vi "UHR-Fleezers Control (host) - 10.2.vi"() -> ()   [LabVIEW 2009] (continued)
        n1205 = local read "AI2 (V)"() -> (w4676:cluster{"Set 1":dbl, "Set 2":dbl})
        n1206 = Or Array Elements(Boolean array=w4678) -> (logical OR=w4679:bool)
        n1207 = Bundle By Name(cluster=w4676, "Set 1"=w4675, "Set 2"=w4674) -> (w4673:cluster{"Set 1":dbl, "Set 2":dbl})
        n1208 = Divide(x=w4673, y=3276.7) -> (x/y=w4672:cluster{"Set 1":dbl, "Set 2":dbl})
        "AI2 (V)" <- w4672
        n1209 = case shown="True" w4679 {
          tunnel: [w4741 w4758] -> w4671
          tunnel: "AI2 to Setpoint" -> [_ w4754]
          tunnel: "Setpoints (V)" -> [w4742 w4757]
          tunnel: w4672 -> [_ w4751]
          frame #0 {
            n1210 = Multiply(x=3276.7, y=w4742) -> (x*y=w4743:cluster{"Set 1":dbl, "Set 2":dbl})
            n1211 = To Word Integer(number=w4743) -> (16bit integer=w4741:cluster{"Set 1":i16, "Set 2":i16})
          }
          frame #1 {
            n1212 = Unbundle By Name(w4751) -> ("Set 1"=w4750:dbl, "Set 2"=w4749:dbl)
            n1213 = Unbundle By Name(w4757) -> ("Set 1"=w4756:dbl, "Set 2"=w4755:dbl)
            n1214 = Unbundle By Name(w4754) -> ("Set 1"=w4753:bool, "Set 2"=w4752:bool)
            n1215 = Select(t=w4750, s=w4753, f=w4756) -> (s? t:f=w4748:dbl)
            n1216 = Select(t=w4749, s=w4752, f=w4755) -> (s? t:f=w4747:dbl)
            n1217 = Bundle By Name(cluster=w4757, "Set 1"=w4748, "Set 2"=w4747) -> (w4745:cluster{"Set 1":dbl, "Set 2":dbl})
            n1218 = Multiply(x=3276.7, y=w4745) -> (x*y=w4746:cluster{"Set 1":dbl, "Set 2":dbl})
            n1219 = local write "Setpoints (V)"(w4745) -> ()
            n1220 = To Word Integer(number=w4746) -> (16bit integer=w4758:cluster{"Set 1":i16, "Set 2":i16})
          }
        }
        n1221 = Unbundle By Name(w4671) -> ("Set 1"=w4670:i16, "Set 2"=w4669:i16)
        n1222 = xnode "Read/Write Control"("FPGA VI Reference In"=w4667, "error in"=w4666, "FB Setpoint Set 1"=w4670, "FB Setpoint Set 2"=w4669) -> ("error out"=w4665:errorcluster)  [unwired: 1 out]
      }
      event #18 {
        n1223 = event-data() -> ()  [unwired: 7 out]
        n1224 = xnode "Read/Write Control"("FPGA VI Reference In"=w4818, "error in"=w4816, "Invert GI"="Invert GI", "Invert GI 2"="Invert GI") -> ("error out"=w4817:errorcluster)  [unwired: 1 out]
      }
      event #19 {
        n1225 = event-data() -> ()  [unwired: 7 out]
        n1226 = local read "Green FB Setpoint (mV)"() -> (w4882:dbl)
        n1227 = local read "Current When FB OFF (%)"() -> (w4885:dbl)
        n1228 = Multiply(x=w4882, y=3.2767) -> (x*y=w4881:dbl)
        n1229 = Multiply(x=w4885, y=655.35) -> (x*y=w4886:dbl)
        n1230 = To Unsigned Word Integer(number=w4886) -> (unsigned 16bit integer=w4884:u16)
        n1231 = local read "Green int current ON count adj"() -> (w4889:u32)
        n1232 = local read "Green FB Gains"() -> (w4888:T14)
        n1233 = local read "Green Laser ON/Interlacing"() -> (w4879:bool)
        n1234 = local read "Green laser mode"() -> (w4878:enum32{"Laser ON", "Laser OFF", "Interlace"})
        n1235 = local read "Green FB On/Off"() -> (w4890:bool)
        n1236 = Equal?(x=w4878, y=enum32{"Laser ON", "Laser OFF", "Interlace"}."Interlace") -> (x = y?=w4876:bool)
        n1237 = Compound Arithmetic op=AND(w4876, w4890, w4879) -> (w4880:bool)
        n1238 = xnode "Read/Write Control"("FPGA VI Reference In"=w4893, "error in"=w4892, "Green FB Setpoint"=w4881, "Green FB On/Off"=w4880, "Current Out"=w4884, "Green int current ON count adj"=w4889, "Green FB Gains"=w4888) -> ("error out"=w4891:errorcluster)  [unwired: 1 out]
      }
      event #20 {
        n1239 = event-data() -> ()  [unwired: 7 out]
        n1240 = case shown="True" "Green Laser ON/Interlacing" {
          tunnel: "Green laser mode" -> [_ w5011]
          tunnel: [enum32{"Laser ON", "Laser OFF", "Interlace"}."Laser OFF" ("Green laser mode") w5011] -> w4999
          tunnel: [FALSE w5007] -> w4998
          frame #0 {
          }
          frame #1 {
            n1241 = local read "Green FB On/Off"() -> (w5008:bool)
            n1242 = Equal?(x=w5011, y=enum32{"Laser ON", "Laser OFF", "Interlace"}."Interlace") -> (x = y?=w5009:bool)
            n1243 = And(x=w5009, y=w5008) -> (x .and. y?=w5007:bool)
          }
        }
        n1244 = xnode "Read/Write Control"("FPGA VI Reference In"=w5004, "error in"=w5002, "Operating Mode"=w4999, "Operating Mode 2"=w4999, "Green FB On/Off"=w4998) -> ("error out"=w5003:errorcluster)  [unwired: 1 out]
      }
      event #21 {
        n1245 = event-data() -> ()  [unwired: 7 out]
        n1246 = local read "Phase Adj. (APD 1 Gate)"() -> (w5087:i16)
        n1247 = Negate(x=w5087) -> (-x=w5095:i16)
        n1248 = Select(t=w5095, s="- phase (APD 1 Gate)", f=w5087) -> (s? t:f=w5094:i16)
        n1249 = Or(x="- phase (APD 1 Gate)", y="+ phase (APD 1 Gate)") -> (x .or. y?=w5090:bool)
        n1250 = xnode "Read/Write Control"("FPGA VI Reference In"=w5097, "error in"=w5096, "Phase count adjustment (APD 1 Gate)"=w5094) -> ("FPGA VI Reference Out"=w5092:T21, "error out"=w5093:errorcluster)
        n1251 = xnode "Read/Write Control"("FPGA VI Reference In"=w5092, "error in"=w5093, "+ phase (APD 1 Gate)"=w5090) -> ("error out"=w5091:errorcluster)  [unwired: 1 out]
      }
      event #22 {
        n1252 = event-data() -> ()  [unwired: 7 out]
        n1253 = local read "Phase Adj. (APD 2 Gate)"() -> (w5171:i16)
        n1254 = Negate(x=w5171) -> (-x=w5179:i16)
        n1255 = Select(t=w5179, s="- phase (APD 2 Gate)", f=w5171) -> (s? t:f=w5178:i16)
        n1256 = Or(x="- phase (APD 2 Gate)", y="+ phase (APD 2 Gate)") -> (x .or. y?=w5174:bool)
        n1257 = xnode "Read/Write Control"("FPGA VI Reference In"=w5181, "error in"=w5180, "Phase count adjustment (APD 2 Gate)"=w5178) -> ("FPGA VI Reference Out"=w5176:T21, "error out"=w5177:errorcluster)
        n1258 = xnode "Read/Write Control"("FPGA VI Reference In"=w5176, "error in"=w5177, "+ phase (APD 2 Gate)"=w5174) -> ("error out"=w5175:errorcluster)  [unwired: 1 out]
      }
      event #23 {
        n1259 = event-data() -> ()  [unwired: 7 out]
        n1260 = local read "Phase Adj. (APD Acq)"() -> (w5257:i16)
        n1261 = Negate(x=w5257) -> (-x=w5263:i16)
        n1262 = Select(t=w5263, s="+ phase (APD Acq)", f=w5257) -> (s? t:f=w5262:i16)
        n1263 = Or(x="+ phase (APD Acq)", y="- phase (APD Acq)") -> (x .or. y?=w5258:bool)
        n1264 = xnode "Read/Write Control"("FPGA VI Reference In"=w5265, "error in"=w5264, "Phase Count Adjustment (APD Acq)"=w5262) -> ("FPGA VI Reference Out"=w5260:T21, "error out"=w5261:errorcluster)
        n1265 = xnode "Read/Write Control"("FPGA VI Reference In"=w5260, "error in"=w5261, "+ phase (APD Acq)"=w5258) -> ("error out"=w5259:errorcluster)  [unwired: 1 out]
      }
      event #24 {
        n1266 = event-data() -> ()  [unwired: 7 out]
        n1267 = Negate(x="Phase adj. (GI)") -> (-x=w5347:i16)
        n1268 = Select(t=w5347, s="+ phase (GI)", f="Phase adj. (GI)") -> (s? t:f=w5346:i16)
        n1269 = Or(x="+ phase (GI)", y="- phase (GI)") -> (x .or. y?=w5342:bool)
        n1270 = xnode "Read/Write Control"("FPGA VI Reference In"=w5349, "error in"=w5348, "Phase count adjustment (GI)"=w5346) -> ("FPGA VI Reference Out"=w5344:T21, "error out"=w5345:errorcluster)
        n1271 = xnode "Read/Write Control"("FPGA VI Reference In"=w5344, "error in"=w5345, "+ phase (GI)"=w5342) -> ("error out"=w5343:errorcluster)  [unwired: 1 out]
      }
      event #25 {
        n1272 = event-data() -> ()  [unwired: 7 out]
        n1273 = Negate(x="Phase adj. (GI) 2") -> (-x=w5431:i16)
        n1274 = Select(t=w5431, s="+ phase (GI) 2", f="Phase adj. (GI) 2") -> (s? t:f=w5430:i16)
        n1275 = Or(x="+ phase (GI) 2", y="- phase (GI) 2") -> (x .or. y?=w5426:bool)
        n1276 = xnode "Read/Write Control"("FPGA VI Reference In"=w5433, "error in"=w5432, "Phase count adjustment (GI) 2"=w5430) -> ("FPGA VI Reference Out"=w5428:T21, "error out"=w5429:errorcluster)
        n1277 = xnode "Read/Write Control"("FPGA VI Reference In"=w5428, "error in"=w5429, "+ phase (GI) 2"=w5426) -> ("error out"=w5427:errorcluster)  [unwired: 1 out]
      }
      event #26 {
        n1278 = event-data() -> ()  [unwired: 7 out]
        n1279 = Negate(x="Phase adj. (Green FB)") -> (-x=w5515:i16)
        n1280 = Select(t=w5515, s="+ phase (Green FB)", f="Phase adj. (Green FB)") -> (s? t:f=w5514:i16)
        n1281 = Or(x="+ phase (Green FB)", y="- phase (Green FB)") -> (x .or. y?=w5510:bool)
        n1282 = xnode "Read/Write Control"("FPGA VI Reference In"=w5517, "error in"=w5516, "Phase count adjustment (Green FB)"=w5514) -> ("FPGA VI Reference Out"=w5512:T21, "error out"=w5513:errorcluster)
        n1283 = xnode "Read/Write Control"("FPGA VI Reference In"=w5512, "error in"=w5513, "+ phase (Green FB)"=w5510) -> ("error out"=w5511:errorcluster)  [unwired: 1 out]
      }
      event #27 {
        n1284 = event-data() -> ()  [unwired: 7 out]
        n1285 = local read "APD Integration Time (s)"() -> (w5591:dbl)
        n1286 = local read "APD Gate ON Count"() -> (w5604:u32)
        n1287 = local read "APD Gate OFF Count"() -> (w5603:u32)
        n1288 = local read "Invert APD Gate"() -> (w5605:bool)
        n1289 = local read "APD Gate"() -> (w5602:enum32{"ON", "OFF", "Interlace"})
        n1290 = Multiply(x=w5591, y=40000000.0) -> (x*y=w5600:dbl)
        n1291 = Reciprocal(x=w5591) -> (1/x=→"APD Acq Rate (Hz)":dbl)
        n1292 = To Unsigned Long Integer(number=w5600) -> (unsigned 32bit integer=w5599:u32)
        n1293 = local read "DMA Update Period (s)"() -> (w5592:dbl)
        n1294 = Divide(x=w5592, y=w5591) -> (x/y=w5595:dbl)
        n1295 = local read "APD 1 AO Mult."() -> (w5597:i16)
        n1296 = local read "APD 2 AO Mult."() -> (w5596:i16)
        n1297 = Multiply(x=2.0, y=w5595) -> (x*y=w5594:dbl)
        n1298 = local write "APD Samples/FIFO Acq."(w5595) -> ()
        n1299 = local write "APD Elements/DMA read"(w5594) -> ()
        n1300 = xnode "Read/Write Control"("FPGA VI Reference In"=w5608, "error in"=w5607, "Invert APD Gate"=w5605, "APD Gate ON Count"=w5604, "APD Gate OFF Count"=w5603, "APD Acq Rate Count"=w5599, "APD Gate Operating Mode"=w5602, "APD 1 AO scale factor"=w5597, "APD 2 AO scale factor"=w5596) -> ("error out"=w5606:errorcluster)  [unwired: 1 out]
      }
      event #28 {
        n1301 = event-data() -> ()  [unwired: 7 out]
        n1302 = xnode "Read/Write Control"("FPGA VI Reference In"=w5765, "error in"=w5763, "Green interlace ON count"="GI Frequency, ON count", "Green interlace OFF count"="GI Frequency, OFF count", "Green interlace ON count 2"="GI Frequency, ON count", "Green interlace OFF count 2"="GI Frequency, OFF count", "Green FB Count"="Green FB Count") -> ("error out"=w5764:errorcluster)  [unwired: 1 out]
      }
      event #29 {
        w5939 = 123.0  # AOM cal (nm/MHz)
        n1303 = event-data() -> ()  [unwired: 7 out]
        n1304 = local read "BD 1 Frequency 1 (MHz)"() -> (w5922:dbl)
        n1305 = local read "AOM X Cal (nm/MHz)"() -> (w5914:dbl)
        n1306 = local read "X RF Frequency Limits (MHz)"() -> (w5926:T16)
        n1307 = local read "Y RF Frequency Limits (MHz)"() -> (w5923:T16)
        n1308 = local read "BD 2 Frequency 1 (MHz)"() -> (w5928:dbl)
        n1309 = Negate(x="Scan Range (nm)") -> (-x=w5892:dbl)
        n1310 = Divide(x=w5892, y=w5914) -> (x/y=w5896:dbl)
        n1311 = Select(t=w5926, s="Scan BD", f=w5923) -> (s? t:f=w5925:T16)
        n1312 = Select(t=w5922, s="Scan BD", f=w5928) -> (s? t:f=w5927:dbl)
        n1313 = Unbundle By Name(w5925) -> ("Maximum"=w5934:dbl, "Minimum"=w5933:dbl)
        n1314 = Add(x=w5896, y=w5927) -> (x+y=w5931:dbl)
        n1315 = Divide(x=w5892, y="Step Size (nm)") -> (x/y=w5911:dbl)
        n1316 = Divide(x="Step Size (nm)", y=w5914) -> (x/y=w5920:dbl)
        n1317 = Absolute Value(x=w5911) -> (abs(x)=w5895:dbl)
        n1318 = Sign(1:w5892) -> (0:w5893:dbl)
        n1319 = In Range and Coerce(upper limit=w5934, x=w5931, lower limit=w5933) -> (coerced(x)=w5930:dbl, In Range?=w5932:bool)
        n1320 = To Unsigned Quad Integer(1:w5895) -> (0:w5910:u64)
        "Scan steps (AOD)" <- w5910
        n1321 = call "IR AOM freq to word.vi"("Frequency In (MHz)"=w5920) -> ("Frequency Word Out (double)"=w5917:dbl)
        n1322 = Multiply(x=w5893, y=w5917) -> (x*y=w5894:dbl)
        n1323 = Subtract(x=w5931, y=w5930) -> (x-y=w5929:dbl)
        n1324 = To Quad Integer(1:w5894) -> (0:w5916:i64)
        "Incr. int (AOD)" <- w5916
        n1325 = Subtract(x=w5896, y=w5929) -> (x-y=w5915:dbl)
        "Scan Range (MHz)" <- w5915
        n1326 = Select(t=w5896, s=w5932, f=w5915) -> (s? t:f=w5935:dbl)
        n1327 = Multiply(x=w5915, y=w5914) -> (x*y=w5913:dbl)
        n1328 = Decrement(x=w5910) -> (x-1=w5963:u64)
        n1329 = Negate(x=w5913) -> (-x=w5909:dbl)
        n1330 = local write "Scan Range (nm)"(w5909) -> ()
        n1331 = Divide(x=w5935, y=w5963) -> (x/y=w5919:dbl)
        "Scan Increment (MHz)" <- w5919
        n1332 = call "IR AOM freq to word.vi"("Frequency In (MHz)"=w5919) -> ("Frequency Word Out (double)"=w5918:dbl)
        n1333 = Divide(x="Step Size (nm)", y="Scan Speed (nm/s)") -> (x/y=w5906:dbl)
        n1334 = To Quad Integer(1:w5918) -> ()  [unwired: 1 out]
        n1335 = local read "Number Interlace Sets"() -> (w5890:u8)
        n1336 = local read "AI Count (ticks)"() -> (w5891:u32)
        n1337 = local read "Total Counts (ticks)"() -> (w5889:u32)
        n1338 = local read "# Samples/trap"() -> (w5921:u32)
        n1339 = Multiply(x=w5891, y=w5890) -> (x*y=w5888:u32)
        n1340 = Divide(x=w5889, y=w5888) -> (x/y=w5887:dbl)
        n1341 = Select(t=w5922, s="Scan BD", f=w5928) -> (s? t:f=w5960:dbl)
        "Initial freq. (MHz)" <- w5960
        n1342 = Add(x=w5935, y=w5960) -> (x+y=→"Final freq. (MHz)":dbl)
        n1343 = Divide(x=w5889, y=40000000.0) -> (x/y=w5905:dbl)
        n1344 = Divide(x=w5906, y=w5905) -> (x/y=w5904:dbl)
        n1345 = To Unsigned Quad Integer(1:w5904) -> (0:w5879:u64)
        n1346 = Quotient & Remainder(x=w5879, y=u64 2) -> (x-y*floor(x/y)=w5883:u64)  [unwired: 1 out]
        n1347 = Equal?(x=w5883, y=u64 0) -> (x = y?=w5881:bool)
        n1348 = Decrement(x=w5879) -> (x-1=w5880:u64)
        n1349 = Select(t=w5879, s=w5881, f=w5880) -> (s? t:f=w5878:u64)
        "Cycles/step (AOD)" <- w5878
        n1350 = xnode "Read/Write Control"("FPGA VI Reference In"=w5971, "error in"=w5970, "Scan steps"=w5910, "Number of scans"="Number of F/B Scans (AOD)", "Cycles per step"=w5878, "Scan freq.  increment"=w5916, "Scan BD"="Scan BD") -> ("error out"=w5969:errorcluster)  [unwired: 1 out]
        n1351 = Multiply(x=w5910, y=w5878) -> (x*y=w5964:u64)
        n1352 = Multiply(x=w5964, y=u64 2) -> (x*y=w5886:u64)
        n1353 = Multiply(x=w5887, y=w5886) -> (x*y=w5885:dbl)
        "Data points/scan (f/b)" <- w5885
        n1354 = Multiply(x=w5885, y="Number of F/B Scans (AOD)") -> (x*y=w5967:dbl)
        "Data points/scans" <- w5967
        n1355 = Divide(x=w5967, y=w5921) -> (x/y=→"N sets should be saved":dbl)
        n1356 = Multiply(x=w5964, y=w5905) -> (x*y=w5903:dbl)
        "Time/Scan (s) (AOD)" <- w5903
        n1357 = Select(t=w5935, s="Scan BD", f=0.0) -> (s? t:f=w5961:dbl)
        n1358 = Select(t=0.0, s="Scan BD", f=w5935) -> (s? t:f=w5957:dbl)
        n1359 = local read "BD 2 Frequency 2 (MHz)"() -> (w5953:dbl)
        n1360 = local read "BD 1 Frequency 2 (MHz)"() -> (w5956:dbl)
        n1361 = Add(x=w5957, y=w5928) -> (x+y=w5954:dbl)
        n1362 = Add(x=w5922, y=w5961) -> (x+y=w5955:dbl)
        n1363 = Multiply(x=w5903, y=2.0) -> (x*y=w5902:dbl)
        n1364 = Multiply(x=w5902, y="Number of F/B Scans (AOD)") -> (x*y=w5899:dbl)
        n1365 = Divide(x=w5899, y=60.0) -> (x/y=→"Time to Finish All (min)":dbl)
        n1366 = Add(x="Trap 2 Bead Size (nm)", y="Trap 1 Bead Size (nm)") -> (x+y=w5943:dbl)
        n1367 = Divide(x=w5943, y=2.0) -> (x/y=w5937:dbl)
        n1368 = Subtract(x=w5954, y=w5953) -> (x-y=w5951:dbl)
        n1369 = Subtract(x=w5955, y=w5956) -> (x-y=w5952:dbl)
        n1370 = local read "Initial delta (MHz)"() -> (w5940:dbl)
        n1371 = Square(x=w5951) -> (x^2=w5950:dbl)
        n1372 = Square(x=w5952) -> (x^2=w5949:dbl)
        n1373 = Add(x=w5949, y=w5950) -> (x+y=w5948:dbl)
        n1374 = Square Root(x=w5948) -> (sqrt(x)=w5947:dbl)
        "Final delta (MHz)" <- w5947
        n1375 = Multiply(x=w5939, y=w5947) -> (x*y=w5946:dbl)
        n1376 = Multiply(x=w5940, y=w5939) -> (x*y=w5938:dbl)
        n1377 = Subtract(x=w5938, y=w5937) -> (x-y=→"Initial sep (nm)":dbl)
        n1378 = Subtract(x=w5946, y=w5937) -> (x-y=→"Final sep (nm)":dbl)
      }
      event #30 {
        n1379 = event-data() -> ()  [unwired: 7 out]
        n1380 = local read "Freq or Amp switch first"() -> (w6058:bool)
        n1381 = local read "Amp switch delay"() -> (w6059:u16)
        n1382 = local read "Freq switch delay"() -> (w6061:u16)
        n1383 = local read "Swap F1 and F2"() -> (w6060:bool)
        n1384 = xnode "Read/Write Control"("FPGA VI Reference In"=w6064, "error in"=w6063, "Freq switch delay"=w6061, "Swap F1 and F2"=w6060, "Amp switch delay"=w6059, "Freq or Amp switch first"=w6058) -> ("error out"=w6062:errorcluster)  [unwired: 1 out]
      }
      event #31 {
        w6161 = 32767.0 ("y")
        n1385 = event-data() -> ()  [unwired: 7 out]
        n1386 = Select(t="Scan lines (y)", s="2D or 1D Scan", f="Number of scans (MCL)") -> (s? t:f=w6166:u64)
        n1387 = Decrement(x="Scan steps (MCL)") -> (x-1=w6182:u64)
        n1388 = Divide(x="Scan Range (V)\n(of steps)", y=w6182) -> (x/y=w6181:dbl)
        "Desired Scan Incr (V)" <- w6181
        n1389 = local read "APD Integration Time (s)"() -> (w6174:dbl)
        n1390 = Multiply(x=w6181, y=w6161) -> (x*y=w6190:dbl)
        n1391 = Divide(x=w6190, y=10.0) -> (x/y=w6180:dbl)
        "Desired incr (int)" <- w6180
        n1392 = local read "Update Count (MCL)"() -> (w6186:u32)
        n1393 = Round Toward -Infinity(1:w6180) -> (0:w6189:dbl)
        n1394 = To Word Integer(number=w6189) -> (16bit integer=w6164:i16)
        "Actual Incr. int (MCL)" <- w6164
        n1395 = Multiply(x=w6174, y=40000000.0) -> (x*y=w6187:dbl)
        n1396 = Divide(x=w6187, y=w6186) -> (x/y=w6185:dbl)
        n1397 = Multiply(x=i16 10, y=w6164) -> (x*y=w6162:i16)
        n1398 = Multiply(x="N APD Samp/step", y=w6185) -> (x*y=w6184:dbl)
        "Cycles/step (MCL)" <- w6184
        n1399 = Divide(x=w6162, y=w6161) -> (x/y=→"Actual MCL Inc (V)":dbl)
        n1400 = Multiply(x="N APD Samp/step", y="Scan steps (MCL)") -> (x*y=w6176:dbl)
        n1401 = local read "APD Samples/FIFO Acq."() -> (w6173:dbl)
        n1402 = Multiply(x=w6176, y=u64 2) -> (x*y=w6175:dbl)
        "Data points/scan (f+b)" <- w6175
        n1403 = Multiply(x=w6175, y=w6166) -> (x*y=w6193:dbl)
        "Data points/scans (MCL)" <- w6193
        n1404 = Multiply(x=w6174, y=w6175) -> (x*y=w6167:dbl)
        "Time/f+b scan (s) (MCL)" <- w6167
        n1405 = Divide(x=w6193, y=w6173) -> (x/y=→"N sets should be saved (MCL)":dbl)
        n1406 = Multiply(x=w6167, y=w6166) -> (x*y=→"Total Time (s)":dbl)
        n1407 = Not(x="Fast Scan Dir") -> (.not. x?=w6171:bool)
        n1408 = xnode "Read/Write Control"("FPGA VI Reference In"=w6197, "error in"=w6196, "Scan steps (MCL)"="Scan steps (MCL)", "Number of scans (MCL)"=w6166, "Cycles per step (MCL)"=w6184, "Scan freq.  increment (MCL)"=w6164, "1D or 2D Scan?"="2D or 1D Scan", "MCL Scan Axis"=w6171, "Cont. Scan (MCL)"="Continuous MCL Scanning") -> ("error out"=w6195:errorcluster)  [unwired: 1 out]
      }
      event #32 {
        w6334 = 1000.0 ("y")
        n1409 = event-data() -> ()  [unwired: 7 out]
        n1410 = local read "Save file name"() -> (w6359:path)
        n1411 = local write "Read Cal"(FALSE ("Read Cal")) -> ()
        n1412 = Strip Path(path=w6359) -> (stripped path=w6358:path)  [unwired: 1 out]
        n1413 = Path To String(path=w6358) -> (string=w6357:string)
        n1414 = Concatenate Strings(w6357, "\\current.cal" ("string")) -> (w6355:string)
        n1415 = String To Path(string=w6355) -> (path=w6354:path)
        n1416 = Open/Create/Replace File(file path (use dialog)=w6354, operation (0:open)=T33."open", access (0:read/write)=enum16{"read/write", "read-only", "write-only"}."read-only") -> (refnum out=w6362:refnum<file>, error out=w6348:errorcluster)  [unwired: 1 in, 3 out]
        n1417 = Deny Access(4:w6348, 7:w6362) -> (0:w6347:errorcluster, 3:w6353:refnum<file>)  [unwired: 1 out]
        n1418 = Read from Binary File(5:0.0, 8:w6347, 9:T34."big-endian, network order" ("byte order (0:big-endian, network order)"), 10:-1 ("count (1)"), 11:w6353) -> (0:w6346:errorcluster, 2:w6344:dbl[], 3:w6349:refnum<file>)  [unwired: 2 out]
        n1419 = Array To Cluster(array=w6344) -> (cluster=w6343:T43)
        n1420 = Unbundle(w6343) -> ("[0]"=w6342:dbl, "[1]"=w6341:dbl, "[2]"=w6340:dbl, "[3]"=w6339:dbl, "[4]"=w6338:dbl, "[5]"=w6337:dbl)
        n1421 = Close File(refnum=w6349, error in=w6346) -> (error out=→"Read cal error":errorcluster)  [unwired: 1 out]
        n1422 = Multiply(x=w6337, y=w6334) -> (x*y=w6335:dbl)
        n1423 = local write "T2 kappa_x (pN/nm)"(w6339) -> ()
        n1424 = local write "T1 kappa_x (pN/nm)"(w6340) -> ()
        n1425 = local write "T1 alpha_x (nm/V)"(w6342) -> ()
        n1426 = local write "T2 alpha_x (nm/V)"(w6341) -> ()
        n1427 = Multiply(x=w6338, y=w6334) -> (x*y=w6336:dbl)
        n1428 = local write "T1 offset_x (mV)"(w6336) -> ()
        n1429 = local write "T2 offset_x (mV)"(w6335) -> ()
      }
      event #33 {
        n1430 = event-data() -> ()  [unwired: 7 out]
        n1431 = local write "MCL Scanning"(FALSE ("MCL Scanning")) -> ()
        n1432 = xnode "Read/Write Control"("FPGA VI Reference In"=w6367, "error in"=w6366, "Abort scan (MCL)"="Abort MCL Scan") -> ("error out"=w6365:errorcluster)  [unwired: 1 out]
      }
      event #34 {
        n1433 = event-data() -> ()  [unwired: 7 out]
        n1434 = xnode "Read/Write Control"("FPGA VI Reference In"=w6408, "error in"=w6407, "MCL count"="Update Count (MCL)") -> ("error out"=w6406:errorcluster)  [unwired: 1 out]
      }
      event #35 {
        n1435 = event-data() -> ()  [unwired: 7 out]
        n1436 = Negate(x="Phase adjust (MCL)") -> (-x=w6453:i16)
        n1437 = Select(t=w6453, s="- phase (MCL)", f="Phase adjust (MCL)") -> (s? t:f=w6451:i16)
        n1438 = Or(x="- phase (MCL)", y="+ phase (MCL)") -> (x .or. y?=w6446:bool)
        n1439 = xnode "Read/Write Control"("FPGA VI Reference In"=w6455, "error in"=w6454, "Phase count adjustment (MCL)"=w6451) -> ("FPGA VI Reference Out"=w6447:T21, "error out"=w6448:errorcluster)
        n1440 = xnode "Read/Write Control"("FPGA VI Reference In"=w6447, "error in"=w6448, "+ phase (MCL)"=w6446) -> ("error out"=w6445:errorcluster)  [unwired: 1 out]
      }
      event #36 {
        n1441 = event-data() -> ()  [unwired: 7 out]
        n1442 = xnode "Read/Write Control"("FPGA VI Reference In"=w6532, "error in"=w6531, "Abort scan"="Abort AOD Scan") -> ("error out"=w6530:errorcluster)  [unwired: 1 out]
      }
      event #37 {
        n1443 = event-data() -> ()  [unwired: 7 out]
        n1444 = xnode "Read/Write Control"("FPGA VI Reference In"=w6573, "error in"=w6572, "Cont. Scan"="Continuous AOD Scanning") -> ("error out"=w6571:errorcluster)  [unwired: 1 out]
      }
      event #38 {
        n1445 = event-data() -> ()  [unwired: 7 out]
        n1446 = call "Create new save file.vi"("Insert"="", "Ext"=".dat" ("string"), "Index In"="Index") -> ("Path Out"=→"Save file name":path, "Index Out"=w6611:dbl)
        "Save index" <- w6611
        n1447 = local write "Index"(w6611) -> ()
      }
      event #39 {
        w6626 = 10.0 ("y")
        w6625 = 32767.0 ("y")
        n1448 = event-data() -> ()  [unwired: 7 out]
        n1449 = local read "AO2"() -> (w6624:dbl)
        n1450 = local read "AO1"() -> (w6621:dbl)
        n1451 = Multiply(x=w6621, y=w6625) -> (x*y=w6620:dbl)
        n1452 = Multiply(x=w6624, y=w6625) -> (x*y=w6623:dbl)
        n1453 = Divide(x=w6620, y=w6626) -> (x/y=w6619:dbl)
        n1454 = Divide(x=w6623, y=w6626) -> (x/y=w6622:dbl)
        n1455 = To Word Integer(number=w6619) -> (16bit integer=w6627:i16)
        n1456 = To Word Integer(number=w6622) -> (16bit integer=w6628:i16)
        n1457 = xnode "Read/Write Control"("FPGA VI Reference In"=w6618, "error in"=w6617, "AO1"=w6627, "AO2"=w6628) -> ("error out"=w6616:errorcluster)  [unwired: 1 out]
      }
      event #40 {
        n1458 = local read "Chemyx Syringe Pump Serial Port"() -> (w6684:refnum<visa-resource-name>)
        n1459 = event-data() -> ()  [unwired: 7 out]
        n1460 = local read "Pump write delay (ms)"() -> (w6685:dbl)
        n1461 = case shown="True" "Inject Pump 1" {
          tunnel: w6685 -> [w6692 w6706]
          tunnel: w6684 -> [w6689 w6705]
          frame #0 {
            n1462 = flat-sequence {
              tunnel: w6689 -> [w6693]
              tunnel: [w6693] -> w6690
              tunnel: w6692 -> [_]
              tunnel: [w6696] -> w6691
              tunnel: w6690 -> [w6696]
              tunnel: w6691 -> [w6697]
              tunnel: [w6697] -> w6687
              tunnel: [w6699] -> w6688
              tunnel: w6687 -> [w6699]
              tunnel: w6688 -> [w6701]
              frame #0 {
                n1463 = call "Write to pump.vi"("string"="enter pump1", "VISA resource name"=w6693) -> ()  [unwired: 1 out]
              }
              frame #1 {
                n1464 = Wait (ms)(milliseconds to wait="Pump pause delay (ms)") -> ()  [unwired: 1 out]
              }
              frame #2 {
                n1465 = call "Write to pump.vi"("string"="stop", "VISA resource name"=w6697) -> ()  [unwired: 1 out]
              }
              frame #3 {
                n1466 = Wait (ms)(milliseconds to wait=u32 500) -> ()  [unwired: 1 out]
              }
              frame #4 {
                n1467 = call "Write to pump.vi"("string"="stop", "VISA resource name"=w6701) -> ()  [unwired: 1 out]
              }
            }
          }
          frame #1 {
            n1468 = flat-sequence {
              tunnel: w6705 -> [w6715]
              tunnel: w6706 -> [w6710]
              tunnel: w6706 -> [w6717]
              tunnel: w6705 -> [w6718]
              tunnel: [w6718] -> w6703
              tunnel: [w6720] -> w6704
              tunnel: w6703 -> [w6720]
              tunnel: w6704 -> [w6722]
              frame #0 {
                n1469 = local read "All Pump Parameters"() -> (w6709:T5)
                n1470 = Unbundle By Name(w6709) -> ("Pump 1"=w6716:T44)
                n1471 = call "Set pump parameters.vi"("Pump write delay (ms)"=w6710, "Volume (uL)"="Ch 2 Inject Volume (uL)", "Rate (uL/h)"="Ch 1 Inject Rate (ul/h)", "Units"=4.0, "Pump #"=1.0, "Pump Parameters In"=w6716, "VISA resource name"=w6715) -> ("Pump Parameters Out"=w6708:T44)  [unwired: 3 in]
                n1472 = Bundle By Name(cluster=w6709, "Pump 1"=w6708) -> (w6707:T5)
                n1473 = local write "All Pump Parameters"(w6707) -> ()
              }
              frame #1 {
                n1474 = Wait (ms)(milliseconds to wait=w6717) -> ()  [unwired: 1 out]
              }
              frame #2 {
                n1475 = call "Write to pump.vi"("string"="start", "VISA resource name"=w6718) -> ()  [unwired: 1 out]
              }
              frame #3 {
                n1476 = Wait (ms)(milliseconds to wait=u32 500) -> ()  [unwired: 1 out]
              }
              frame #4 {
                n1477 = call "Write to pump.vi"("string"="start", "VISA resource name"=w6722) -> ()  [unwired: 1 out]
              }
            }
          }
        }
      }
      event #41 {
        n1478 = event-data() -> ()  [unwired: 7 out]
        n1479 = local read "Pump write delay (ms)"() -> (w6725:dbl)
        n1480 = case shown="False" "Inject Pump 3" {
          tunnel: w6725 -> [w6732 w6746]
          tunnel: "Chemyx Syringe Pump Serial Port" -> [w6729 w6745]
          frame #0 {
            n1481 = flat-sequence {
              tunnel: w6729 -> [w6733]
              tunnel: [w6733] -> w6730
              tunnel: w6732 -> [_]
              tunnel: [w6736] -> w6731
              tunnel: w6730 -> [w6736]
              tunnel: w6731 -> [w6737]
              tunnel: [w6737] -> w6727
              tunnel: [w6739] -> w6728
              tunnel: w6727 -> [w6739]
              tunnel: w6728 -> [w6741]
              frame #0 {
                n1482 = call "Write to pump.vi"("string"="enter pump3", "VISA resource name"=w6733) -> ()  [unwired: 1 out]
              }
              frame #1 {
                n1483 = local read "Pump pause delay (ms)"() -> (w6735:u32)
                n1484 = Wait (ms)(milliseconds to wait=w6735) -> ()  [unwired: 1 out]
              }
              frame #2 {
                n1485 = call "Write to pump.vi"("string"="stop", "VISA resource name"=w6737) -> ()  [unwired: 1 out]
              }
              frame #3 {
                n1486 = Wait (ms)(milliseconds to wait=u32 0) -> ()  [unwired: 1 out]
              }
              frame #4 {
                n1487 = call "Write to pump.vi"("string"="stop", "VISA resource name"=w6741) -> ()  [unwired: 1 out]
              }
            }
          }
          frame #1 {
            n1488 = flat-sequence {
              tunnel: w6745 -> [w6755]
              tunnel: w6746 -> [w6750]
              tunnel: w6746 -> [w6757]
              tunnel: w6745 -> [w6758]
              tunnel: [w6758] -> w6743
              tunnel: [w6761] -> w6744
              tunnel: w6743 -> [w6761]
              tunnel: w6744 -> [w6762]
              frame #0 {
                n1489 = local read "All Pump Parameters"() -> (w6749:T5)
                n1490 = Unbundle By Name(w6749) -> ("Pump 3"=w6756:T44)
                n1491 = call "Set pump parameters.vi"("Pump write delay (ms)"=w6750, "Volume (uL)"="Ch 3 Inject Volume (uL)", "Rate (uL/h)"="Ch 3 Inject Rate (ul/h)", "Units"=4.0, "Pump #"=3.0, "Pump Parameters In"=w6756, "VISA resource name"=w6755) -> ("Pump Parameters Out"=w6748:T44)  [unwired: 3 in]
                n1492 = Bundle By Name(cluster=w6749, "Pump 3"=w6748) -> (w6747:T5)
                n1493 = local write "All Pump Parameters"(w6747) -> ()
              }
              frame #1 {
                n1494 = Wait (ms)(milliseconds to wait=w6757) -> ()  [unwired: 1 out]
              }
              frame #2 {
                n1495 = call "Write to pump.vi"("string"="start", "VISA resource name"=w6758) -> ()  [unwired: 1 out]
              }
              frame #3 {
                n1496 = Wait (ms)(milliseconds to wait=u32 500) -> ()  [unwired: 1 out]
              }
              frame #4 {
                n1497 = call "Write to pump.vi"("string"="start", "VISA resource name"=w6762) -> ()  [unwired: 1 out]
              }
            }
          }
        }
      }
      event #42 {
        n1498 = event-data() -> ()  [unwired: 7 out]
        n1499 = local read "Pump write delay (ms)"() -> (w6766:dbl)
        n1500 = flat-sequence {
          tunnel: w6764 -> [w6779]
          tunnel: w6766 -> [w6775]
          tunnel: "Inject Pump 2" -> [_]
          tunnel: w6766 -> [w6781]
          tunnel: w6764 -> [w6782]
          frame #0 {
            n1501 = local read "All Pump Parameters"() -> (w6774:T5)
            n1502 = Multiply(x=60.0, y="Flush Center Ch Rate (ul/m)") -> (x*y=w6771:dbl)
            n1503 = Unbundle By Name(w6774) -> ("Pump 2"=w6780:T44)
            n1504 = call "Set pump parameters.vi"("Pump write delay (ms)"=w6775, "Volume (uL)"="Flush Center Ch Volume (uL)", "Rate (uL/h)"=w6771, "Units"=3.0, "Pump #"=2.0, "Pump Parameters In"=w6780, "VISA resource name"=w6779) -> ("Pump Parameters Out"=w6773:T44)  [unwired: 3 in]
            n1505 = Bundle By Name(cluster=w6774, "Pump 2"=w6773) -> (w6772:T5)
            n1506 = local write "All Pump Parameters"(w6772) -> ()
            n1507 = Add(x="Flush Center Ch Volume (uL)", y="Total Volume\nFlushed (uL)") -> (x+y=w6768:dbl)
            n1508 = local write "Total Volume\nFlushed (uL)"(w6768) -> ()
          }
          frame #1 {
            n1509 = Wait (ms)(milliseconds to wait=w6781) -> ()  [unwired: 1 out]
          }
          frame #2 {
            n1510 = call "Write to pump.vi"("string"="start", "VISA resource name"=w6782) -> ()  [unwired: 1 out]
          }
        }
        n1511 = local read "Chemyx Syringe Pump Serial Port"() -> (w6764:refnum<visa-resource-name>)
      }
      event #43 {
        n1512 = event-data() -> ()  [unwired: 7 out]
        n1513 = Select(t="run" ("string"), s="Sample Channel Flow", f="stop" ("string")) -> (s? t:f=w6784:string)
        n1514 = Concatenate Strings(w6784, "\r") -> (w6788:string)
        n1515 = VISA Write(VISA resource name=w6790, write buffer=w6788) -> ()  [unwired: 1 in, 3 out]
      }
      event #44 {
        n1516 = event-data() -> ()  [unwired: 7 out]
        n1517 = Not(x="Flip Green Filter") -> (.not. x?=w6791:bool)
        n1518 = local write "Flip Green Filter"(w6791) -> ()
        n1519 = flat-sequence {
          tunnel: w6799 -> [w6804]
          tunnel: w6798 -> [w6803]
          tunnel: [w6801] -> w6796
          tunnel: [w6800] -> w6795
          tunnel: [w6843] -> w6794
          tunnel: w6796 -> [w6843]
          tunnel: [w6842] -> w6793
          tunnel: w6795 -> [w6842]
          tunnel: w6794 -> [w6847]
          tunnel: w6793 -> [w6846]
          tunnel: [w6845] -> w6797
          frame #0 {
            n1520 = xnode "Read/Write Control"("FPGA VI Reference In"=w6804, "error in"=w6803, "Green Filter Flipper"=TRUE) -> ("FPGA VI Reference Out"=w6801:T21, "error out"=w6800:errorcluster)
          }
          frame #1 {
            n1521 = Wait (ms)(milliseconds to wait=u32 100) -> ()  [unwired: 1 out]
          }
          frame #2 {
            n1522 = xnode "Read/Write Control"("FPGA VI Reference In"=w6847, "error in"=w6846, "Green Filter Flipper"=FALSE) -> ("error out"=w6845:errorcluster)  [unwired: 1 out]
          }
        }
      }
      event #45 {
        n1523 = event-data() -> ()  [unwired: 7 out]
        n1524 = local read "Pump 1 contents"() -> (→"Pump 1 cont disp":string)
        n1525 = local read "Pump 3 contents"() -> (→"Pump 3 cont disp":string)
      }
      event #46 {
        n1526 = event-data() -> ()  [unwired: 7 out]
        n1527 = xnode "Read/Write Control"("FPGA VI Reference In"=w6890, "error in"=w6889, "Trap Pos. FB Reset"="Reset Trap Pos. FB") -> ()  [unwired: 2 out]
      }
      event #47 {
        n1528 = event-data() -> ()  [unwired: 7 out]
        n1529 = xnode "Read/Write Control"("FPGA VI Reference In"=w6930, "error in"=w6929, "Force feedback"="Trap Pos. FB ON") -> ()  [unwired: 2 out]
      }
      event #48 {
        n1530 = event-data() -> ()  [unwired: 7 out]
        n1531 = xnode "Read/Write Control"("FPGA VI Reference In"=w6976, "error in"=w6975, "Trap Pos. FB Range"="Trap Pos. FB Range", "Trap Pos. FB Gains"="Trap Pos. FB Gains", "Trap Pos. FB Mult Factor"="Trap Pos. FB Mult Factor", "Trap Pos. FB Offset Factor"="Trap Pos. FB Offset Factor", "Trap Pos FB Negate Action"="Trap Pos FB Negate Action", "Trap Pos FB Monitor T1 or T2"="Trap Pos FB Monitor\nT1 or T2", "AI1 X Scale"="Trap Pos. AI1 X Pre-scale") -> ()  [unwired: 2 out]
      }
      event #49 {
        n1532 = event-data() -> ()  [unwired: 7 out]
        n1533 = xnode "Read/Write Control"("FPGA VI Reference In"=w7112, "error in"=w7111, "Trap Pos. FB SP"="Trap Pos FB SP") -> ()  [unwired: 2 out]
      }
      event #50 {
        n1534 = event-data() -> ()  [unwired: 7 out]
        n1535 = local read "Trap Pos FB Monitor\nT1 or T2"() -> (w7165:bool)
        n1536 = local read "Trap X AI1 (DMA)"() -> (w7168:T13)
        n1537 = local read "Trap X (AI1)"() -> (w7171:T10)
        n1538 = local write "Set SP to Reading"(FALSE ("Set SP to Reading")) -> ()
        n1539 = Unbundle By Name(w7171) -> ("Trap 1"=w7170:fxp<+/-,16,1>, "Trap 2"=w7169:fxp<+/-,16,1>)
        n1540 = Unbundle By Name(w7168) -> ("Set 1"=w7167:fxp<+/-,16,1>, "Set 2"=w7166:fxp<+/-,16,1>)
        n1541 = Select(t=w7170, s=w7165, f=w7169) -> (s? t:f=w7164:fxp<+/-,16,1>)
        n1542 = Select(t=w7167, s=w7165, f=w7166) -> (s? t:f=w7163:fxp<+/-,16,1>)
        n1543 = Not(x="Set SP Using...") -> (.not. x?=w7158:bool)
        n1544 = Select(t=w7164, s=w7158, f=w7163) -> (s? t:f=w7159:fxp<+/-,16,1>)
        n1545 = xnode "Read/Write Control"("FPGA VI Reference In"=w7161, "error in"=w7160, "Trap Pos. FB SP"=w7159) -> ()  [unwired: 2 out]
        n1546 = local write "Trap Pos FB SP"(w7159) -> ()
      }
      event #51 {
        n1547 = event-data() -> ()  [unwired: 7 out]
        n1548 = Scale By Power Of 2(n="Trap Pos. FB Out Scale 2^n", x=ext 1.0) -> (x*2^n=w7216:ext)
        n1549 = property on="Trap Pos. FB Mult Factor" class="DigNum (strict)"("Val(Sgnl)"=w7216) -> ()  [unwired: 2 in, 2 out]
      }
      event #52 {
        n1550 = event-data() -> ()  [unwired: 7 out]
        n1551 = xnode "Read/Write Control"("FPGA VI Reference In"=w7221, "error in"=w7220, "Trap Pos FB Int Count"="Trap Pos FB Int Count") -> ()  [unwired: 2 out]
      }
    }
    "error out 2" <- w4006
    n1552 = node-c288() -> ()  [unwired: 2 out]
  }
  n1553 = timed-loop "Mouse control: trap position (AOM deflection), set confocal spot from image" {
    tunnel: [w7259] -> w156
    tunnel: w8 -> [w7258]
    timing: w52 -> [_]
    timing-out: [_] -> w51
    stop <- w7259 stop-if-true
    n1554 = node-c288() -> ()  [unwired: 2 out]
    n1555 = event shown="[0] \"Pane\": Mouse Down" {
      selector: _ -> [_ _]
      dyn-events: _ -> [_ _]
      timeout: _ -> [_ _]
      tunnel: w7258 -> [w7262 _]
      event #0 {
        n1556 = event-data() -> ("Time"=w7264:u32, "Coords"=w7263:T7, "Button"=w7265:u16)  [unwired: 6 out]
        n1557 = case shown="1" w7265 {
          tunnel: w7264 -> [_ _ w7368]
          tunnel: w7263 -> [_ w7302 w7366]
          tunnel: w7262 -> [_ _ w7364]
          frame #0 {
          }
          frame #1 {
            n1558 = property on="APD 2" class="ImageControl"() -> ("Displayed Image Position"=w7272:cluster{"Left":i32, "Top":i32})  [unwired: 2 in, 2 out]
            n1559 = property on="APD 1" class="ImageControl"() -> ("Displayed Image Position"=w7301:cluster{"Left":i32, "Top":i32})  [unwired: 2 in, 2 out]
            n1560 = property on="Detection Laser X" class="ImageControl"() -> ("Displayed Image Position"=w7298:cluster{"Left":i32, "Top":i32})  [unwired: 2 in, 2 out]
            n1561 = property on="Detection Laser Y" class="ImageControl"() -> ("Displayed Image Position"=w7297:cluster{"Left":i32, "Top":i32})  [unwired: 2 in, 2 out]
            n1562 = property on="APD 2" class="ImageControl"() -> ("Displayed Image Size"=w7271:cluster{"Width":u32, "Height":u32})  [unwired: 2 in, 2 out]
            n1563 = property on="APD 1" class="ImageControl"() -> ("Displayed Image Size"=w7299:cluster{"Width":u32, "Height":u32})  [unwired: 2 in, 2 out]
            n1564 = property on="Detection Laser X" class="ImageControl"() -> ("Displayed Image Size"=w7300:cluster{"Width":u32, "Height":u32})  [unwired: 2 in, 2 out]
            n1565 = property on="Detection Laser Y" class="ImageControl"() -> ("Displayed Image Size"=w7296:cluster{"Width":u32, "Height":u32})  [unwired: 2 in, 2 out]
            n1566 = Unbundle By Name(w7271) -> ("Width"=w7268:u32, "Height"=w7267:u32)
            n1567 = Unbundle By Name(w7272) -> ("Left"=w7270:i32, "Top"=w7269:i32)
            n1568 = Unbundle By Name(w7299) -> ("Width"=w7293:u32, "Height"=w7292:u32)
            n1569 = Unbundle By Name(w7300) -> ("Width"=w7289:u32, "Height"=w7288:u32)
            n1570 = Unbundle By Name(w7296) -> ("Width"=w7285:u32, "Height"=w7284:u32)
            n1571 = Unbundle By Name(w7301) -> ("Left"=w7295:i32, "Top"=w7294:i32)
            n1572 = Unbundle By Name(w7298) -> ("Left"=w7291:i32, "Top"=w7290:i32)
            n1573 = Unbundle By Name(w7297) -> ("Left"=w7287:i32, "Top"=w7286:i32)
            n1574 = Bundle("Left"=w7270, "Top"=w7269, "Width"=w7268, "Height"=w7267) -> (w7266:T45)  [unwired: 1 in]
            n1575 = Bundle("Left"=w7295, "Top"=w7294, "Width"=w7293, "Height"=w7292) -> (w7283:T45)  [unwired: 1 in]
            n1576 = Bundle("Left"=w7291, "Top"=w7290, "Width"=w7289, "Height"=w7288) -> (w7282:T45)  [unwired: 1 in]
            n1577 = Bundle("Left"=w7287, "Top"=w7286, "Width"=w7285, "Height"=w7284) -> (w7281:T45)  [unwired: 1 in]
            n1578 = Build Cluster Array(w7266, w7283, w7282, w7281) -> (w7280:T46)
            n1579 = for {
              tunnel: w7302 -> [w7313]
              tunnel: w7280 -> [w7314] mode=indexing
              shift-right: [w7311] -> w7278
              shift-left: TRUE -> [w7312]
              shift-right: [w7310] -> w7276
              shift-left: _ -> [w7306]
              shift-right: [w7309] -> w7275
              shift-left: _ -> [w7305]
              shift-right: [w7308] -> w7274
              shift-left: _ -> [w7304]
              shift-right: [w7307] -> w7273
              shift-left: _ -> [w7303]
              n1580 = case shown="True" w7312 {
                selector: w7312 -> [w7319 _]
                tunnel: w7314 -> [_ w7328]
                tunnel: w7313 -> [_ w7326]
                tunnel: [w7319 w7324] -> w7311
                tunnel: [w7318 w7323] -> w7310
                tunnel: [w7317 w7322] -> w7309
                tunnel: [w7316 w7321] -> w7308
                tunnel: [w7315 w7320] -> w7307
                tunnel: w7306 -> [w7318 _]
                tunnel: w7305 -> [w7317 _]
                tunnel: w7304 -> [w7316 _]
                tunnel: w7303 -> [w7315 _]
                frame #0 {
                }
                frame #1 {
                  n1581 = Unbundle(w7328) -> (w7327:T45)
                  n1582 = call "isclickinwindow.vi"("Image Param"=w7327, "Point32"=w7326) -> ("4 Y"=w7320:i32, "3 Height"=w7321:i32, "2 X"=w7322:i32, "1 Width"=w7323:i32, "In image?"=w7325:bool)  [unwired: 1 in]
                  n1583 = Not(x=w7325) -> (.not. x?=w7324:bool)
                }
              }
            }
            n1584 = Not(x=w7278) -> (.not. x?=w7277:bool)
            n1585 = case shown="True" w7277 {
              tunnel: w7275 -> [_ w7341]
              tunnel: w7273 -> [_ w7340]
              tunnel: w7276 -> [_ w7339]
              tunnel: w7274 -> [_ w7338]
              frame #0 {
              }
              frame #1 {
                w7334 = FALSE ("Get Point")
                n1586 = local read "Scan lines (y)"() -> (w7343:u64)
                n1587 = local read "Actual MCL Inc (V)"() -> (w7335:dbl)
                n1588 = local read "Scan steps (MCL)"() -> (w7342:u64)
                n1589 = Divide "Y Pix/step"(x=w7338, y=w7343) -> (x/y=w7350:dbl)
                n1590 = Divide "Y V/pix"(x=w7335, y=w7350) -> (x/y=w7349:dbl)
                n1591 = Divide "Y half step offset"(x=w7335, y=2.0) -> (x/y=w7351:dbl)
                n1592 = Divide "X pix/step"(x=w7339, y=w7342) -> (x/y=w7348:dbl)
                n1593 = Negate(x=w7351) -> (-x=w7352:dbl)
                n1594 = local read "Initial Y"() -> (w7358:dbl)
                n1595 = Multiply(x=w7340, y=w7349) -> (x*y=w7359:dbl)
                n1596 = Divide "X half step offset"(x=w7335, y=2.0) -> (x/y=w7345:dbl)
                n1597 = Divide "X V/pix"(x=w7335, y=w7348) -> (x/y=w7347:dbl)
                n1598 = Multiply(x=w7335, y=w7342) -> (x*y=w7354:dbl)
                n1599 = Compound Arithmetic op=ADD(w7352, w7359, w7358) -> (w7336:dbl)
                "Pointer Y (V)" <- w7336
                n1600 = Multiply(x=w7347, y=w7341) -> (x*y=w7356:dbl)
                n1601 = Negate(x=w7345) -> (-x=w7344:dbl)
                n1602 = local read "Initial X"() -> (w7357:dbl)
                n1603 = Negate(x=w7356) -> (-x=w7355:dbl)
                n1604 = Compound Arithmetic op=ADD(w7344, w7354, w7357, w7355) -> (w7337:dbl)
                "Pointer X (V)" <- w7337
                n1605 = Or(x="Set X Only", y="Set Confocal Spot (X-Y)") -> (x .or. y?=w7330:bool)
                n1606 = Or(x="Set Confocal Spot (X-Y)", y="Set Y Only") -> (x .or. y?=w7329:bool)
                n1607 = case shown="True" w7330 {
                  tunnel: w7337 -> [_ w7360]
                  frame #0 {
                  }
                  frame #1 {
                    n1608 = property on="AO2" class="Slide (strict)"("Val(Sgnl)"=w7360) -> ()  [unwired: 2 in, 2 out]
                  }
                }
                n1609 = case shown="True" w7329 {
                  tunnel: w7336 -> [_ w7361]
                  frame #0 {
                  }
                  frame #1 {
                    n1610 = property on="AO1" class="Slide (strict)"("Val(Sgnl)"=w7361) -> ()  [unwired: 2 in, 2 out]
                  }
                }
                n1611 = local write "Set Confocal Spot (X-Y)"(w7334) -> ()
                n1612 = local write "Set X Only"(w7334) -> ()
                n1613 = local write "Set Y Only"(w7334) -> ()
              }
            }
          }
          frame #2 {
            n1614 = local read "BD 2 Frequency 1 (MHz)"() -> (w7362:dbl)
            n1615 = local read "BD 1 Frequency 1 (MHz)"() -> (w7363:dbl)
            n1616 = local write "Manipulating Trap"(TRUE ("Manipulating Trap")) -> ()
            n1617 = local write "Coords"(T7 {"Horizontal"=0, "Vertical"=0} ("Coords")) -> ()
            n1618 = while {
              tunnel: w7368 -> [w7373]
              tunnel: w7366 -> [w7372]
              tunnel: w7364 -> [w7371]
              tunnel: w7363 -> [w7370]
              tunnel: w7362 -> [w7369]
              stop <- w7374 stop-if-true
              n1619 = event shown="[0] \"Pane\": Mouse Move" {
                selector: _ -> [_ _]
                dyn-events: _ -> [_ _]
                timeout: _ -> [_ _]
                tunnel: ["Force Manip Abort" w7438] -> w7374
                tunnel: w7373 -> [w7381 _]
                tunnel: w7372 -> [w7379 _]
                tunnel: w7371 -> [w7378 _]
                tunnel: w7370 -> [w7377 _]
                tunnel: w7369 -> [w7376 _]
                event #0 {
                  n1620 = event-data() -> ("Time"=w7382:u32, "Coords"=w7383:T7)  [unwired: 3 out]
                  n1621 = Less?(x=w7382, y=w7381) -> (x < y?=w7380:bool)
                  n1622 = case "Makes sure old motion events prior to mouse click aren't used" shown="False" w7380 {
                    tunnel: w7383 -> [w7425 _]
                    tunnel: w7379 -> [w7426 _]
                    tunnel: w7378 -> [w7403 _]
                    tunnel: w7377 -> [w7399 _]
                    tunnel: w7376 -> [w7398 _]
                    frame #0 {
                      n1623 = Subtract(x=w7425, y=w7426) -> (x-y=w7424:T7)
                      "Coords" <- w7424
                      n1624 = local read "Y RF Frequency Limits (MHz)"() -> (w7384:T16)
                      n1625 = To Double Precision Float(number=w7424) -> (double precision float=w7423:cluster{"Horizontal":dbl, "Vertical":dbl})
                      n1626 = Multiply(x=cluster{"Horizontal":dbl, "Vertical":dbl} {"Horizontal"=-1.0, "Vertical"=1.0}, y="Manipulation Scaling") -> (x*y=w7419:cluster{"Horizontal":dbl, "Vertical":dbl})
                      n1627 = local read "X RF Frequency Limits (MHz)"() -> (w7385:T16)
                      n1628 = Multiply(x=w7423, y=w7419) -> (x*y=w7421:cluster{"Horizontal":dbl, "Vertical":dbl})
                      n1629 = Unbundle By Name(w7421) -> ("Horizontal"=w7416:dbl, "Vertical"=w7420:dbl)
                      n1630 = Unbundle By Name(w7384) -> ("Maximum"=w7387:dbl, "Minimum"=w7386:dbl)
                      n1631 = Boolean To (0,1)(Boolean="Manip. X?") -> (0, 1=w7414:i16)
                      n1632 = Boolean To (0,1)(Boolean="Manip. Y?") -> (0, 1=w7411:i16)
                      n1633 = Multiply(x=w7420, y=w7411) -> (x*y=w7413:dbl)
                      n1634 = Multiply(x=w7414, y=w7416) -> (x*y=w7417:dbl)
                      n1635 = local read "BD 1 Frequency 2 (MHz)"() -> (w7401:dbl)
                      n1636 = Unbundle By Name(w7385) -> ("Maximum"=w7389:dbl, "Minimum"=w7388:dbl)
                      n1637 = local read "BD 2 Frequency 2 (MHz)"() -> (w7400:dbl)
                      n1638 = Add(x=w7398, y=w7413) -> (x+y=w7391:dbl)
                      n1639 = Add(x=w7399, y=w7417) -> (x+y=w7393:dbl)
                      n1640 = In Range and Coerce(upper limit=w7389, x=w7393, lower limit=w7388) -> (coerced(x)=w7392:dbl)  [unwired: 1 out]
                      n1641 = In Range and Coerce(upper limit=w7387, x=w7391, lower limit=w7386) -> (coerced(x)=w7390:dbl)  [unwired: 1 out]
                      n1642 = Subtract(x=w7392, y=w7401) -> (x-y=w7410:dbl)
                      n1643 = Subtract(x=w7390, y=w7400) -> (x-y=w7409:dbl)
                      n1644 = Square(x=w7410) -> (x^2=w7408:dbl)
                      n1645 = Square(x=w7409) -> (x^2=w7407:dbl)
                      n1646 = Add(x=w7408, y=w7407) -> (x+y=w7406:dbl)
                      n1647 = Square Root(x=w7406) -> (sqrt(x)=w7402:dbl)
                      n1648 = In Range and Coerce(upper limit="Limit Max (MHz)", x=w7402, lower limit="Limit Min (MHz)") -> (In Range?=w7395:bool)  [unwired: 1 out]
                      n1649 = Not(x="Limits Enable") -> (.not. x?=w7394:bool)
                      n1650 = Or(x=w7395, y=w7394) -> (x .or. y?=w7396:bool)
                      n1651 = case shown="True" w7396 {